vi "LP_Rx_and_BMon.vi"(0 "Rx":waveform(dbl)={"t0"=timestamp(3771075609.2144814 s since 1904-01-01), "dt"=4.999999999999579e-07, "Y"=array[336000 elements], "attributes"=variant("NI_ChannelName"=variant(string "H1/ai7"), "NI_UnitDescription"=variant(string "Volts"))}, 1 "Bias":waveform(dbl)={"t0"=timestamp(3771075609.3975773 s since 1904-01-01), "dt"=4.999999999999579e-07, "Y"=array[336000 elements], "attributes"=variant("NI_ChannelName"=variant(string "H1/ai5"), "NI_UnitDescription"=variant(string "Volts"))}, 2 "BMon":waveform(dbl)={"t0"=timestamp(3771075609.3975773 s since 1904-01-01), "dt"=4.999999999999579e-07, "Y"=array[336000 elements], "attributes"=variant("NI_ChannelName"=variant(string "H1/ai5"), "NI_UnitDescription"=variant(string "Volts"))}, 3 "BaselineSig":dbl[](array[numeric])=array[336000 elements]) -> (5 "RxBaselineSub":dbl[](graph), 6 "RX_Smooth":dbl[](array[numeric]), 7 "BiasSmooth":dbl[](array[numeric]), 8 "BMon Smooth":dbl[](array[numeric]), 9 "Bias Reconstructed":dbl[](array[numeric]))   [LabVIEW 2021]
uses:
  <vilib>/Analysis/baseanly.llb/Mean (DBL).vi
  <vilib>/Waveform/WDTOps.llb/WDT Number of Waveform Samples DBL.vi
  MPS_global_variables.vi
  <vilib>/measure/macond.llb/Continuous Waveform Convolution for 1 Chan.vi
  <vilib>/measure/matone.llb/Extract Single Tone Information 1 Chan.vi
  <vilib>/measure/NI_MAPro.lvlib
  <vilib>/Analysis/NI_AALBase.lvlib
  <vilib>/measure/NI_MABase.lvlib
panel:
  out "x/y":dbl=168000.0
  out "detected amplitude 2":dbl=0.10391083925713944 format="%.2p"
  out "Bias_IMon_Amps_MeanSub":waveform(dbl)(graph)={"t0"=timestamp(3771075609.3975773 s since 1904-01-01), "dt"=4.999999999999579e-07, "Y"=[], "attributes"=variant("NI_ChannelName"=variant(string "H1/ai5"), "NI_UnitDescription"=variant(string "Volts"))}
  in  "Bias Reconstruct Phase offset":dbl=-4.0 format="%#_13g"
  in  "index":i32
  out "BMon In":waveform(dbl)(graph)={"t0"=timestamp(3771075609.3975773 s since 1904-01-01), "dt"=4.999999999999579e-07, "Y"=array[336000 elements], "attributes"=variant("NI_ChannelName"=variant(string "H1/ai5"), "NI_UnitDescription"=variant(string "Volts"))}
  out "XY Graph":cluster{"Y":dbl[], "Y":dbl[]}[](graph)
  out "Bias_Reconstructed":dbl[](graph)
  out "BMon Smooth":dbl[](graph)
  out "Bias Smooth":dbl[](graph)
  out "Rx Smooth Graph":dbl[](graph)
  in  "advanced search":T1={"approx freq. (optional)"=-1.0, "search (+/- % of Fsampl.)"=5.0} {"search (+/- % of Fsampl.)" format="%0.2p"; "approx freq. (optional)" format="%0.2p"}
  in  "Crop Bias Periods":dbl=5.0
  out "Length_Conv":dbl=84.0
  out "Bias mT/V":dbl=249.6
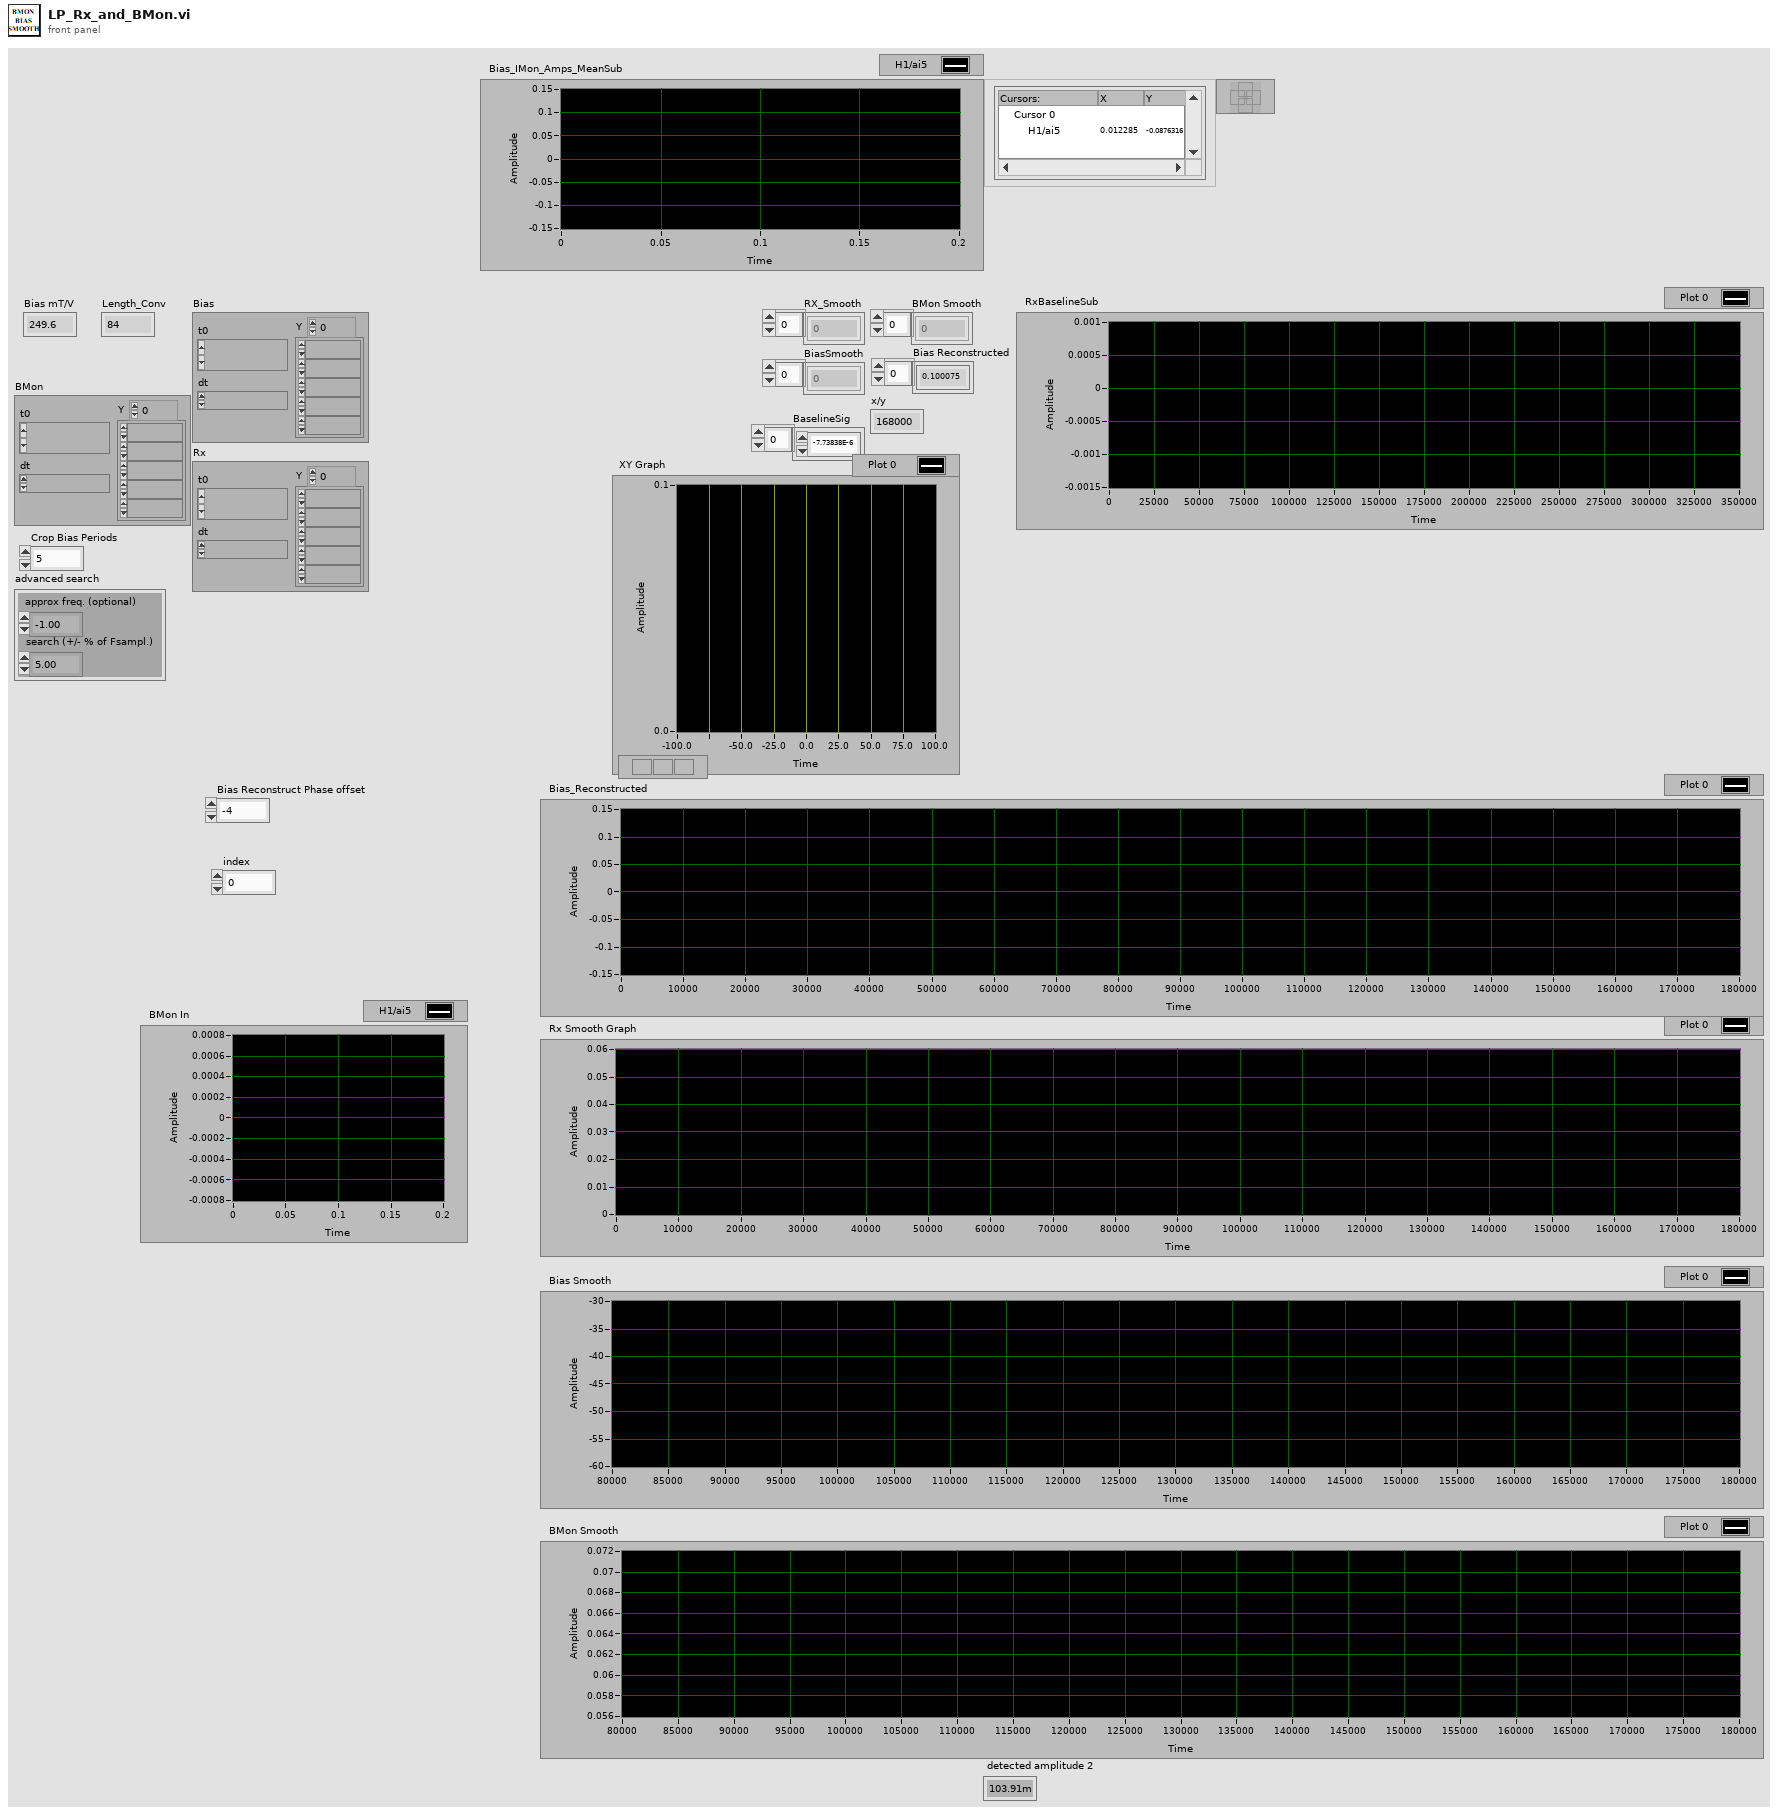
[diagram p1: front panel]
types:
  T1 = cluster{"approx freq. (optional)":dbl, "search (+/- % of Fsampl.)":dbl}
  T2 = cluster{"sample rate":dbl, "Tx freq":dbl, "Tx amp":dbl, "Tx cycles\nSpectroscopy":dbl, "Bias amp":dbl, "Bias freq":dbl, "Receive range":dbl, "Bias Periods\nMagnetometry":dbl, "Tx Freq Division Factor":dbl, "Drive Periods per Bias":dbl, "TX harmonics":dbl[]}
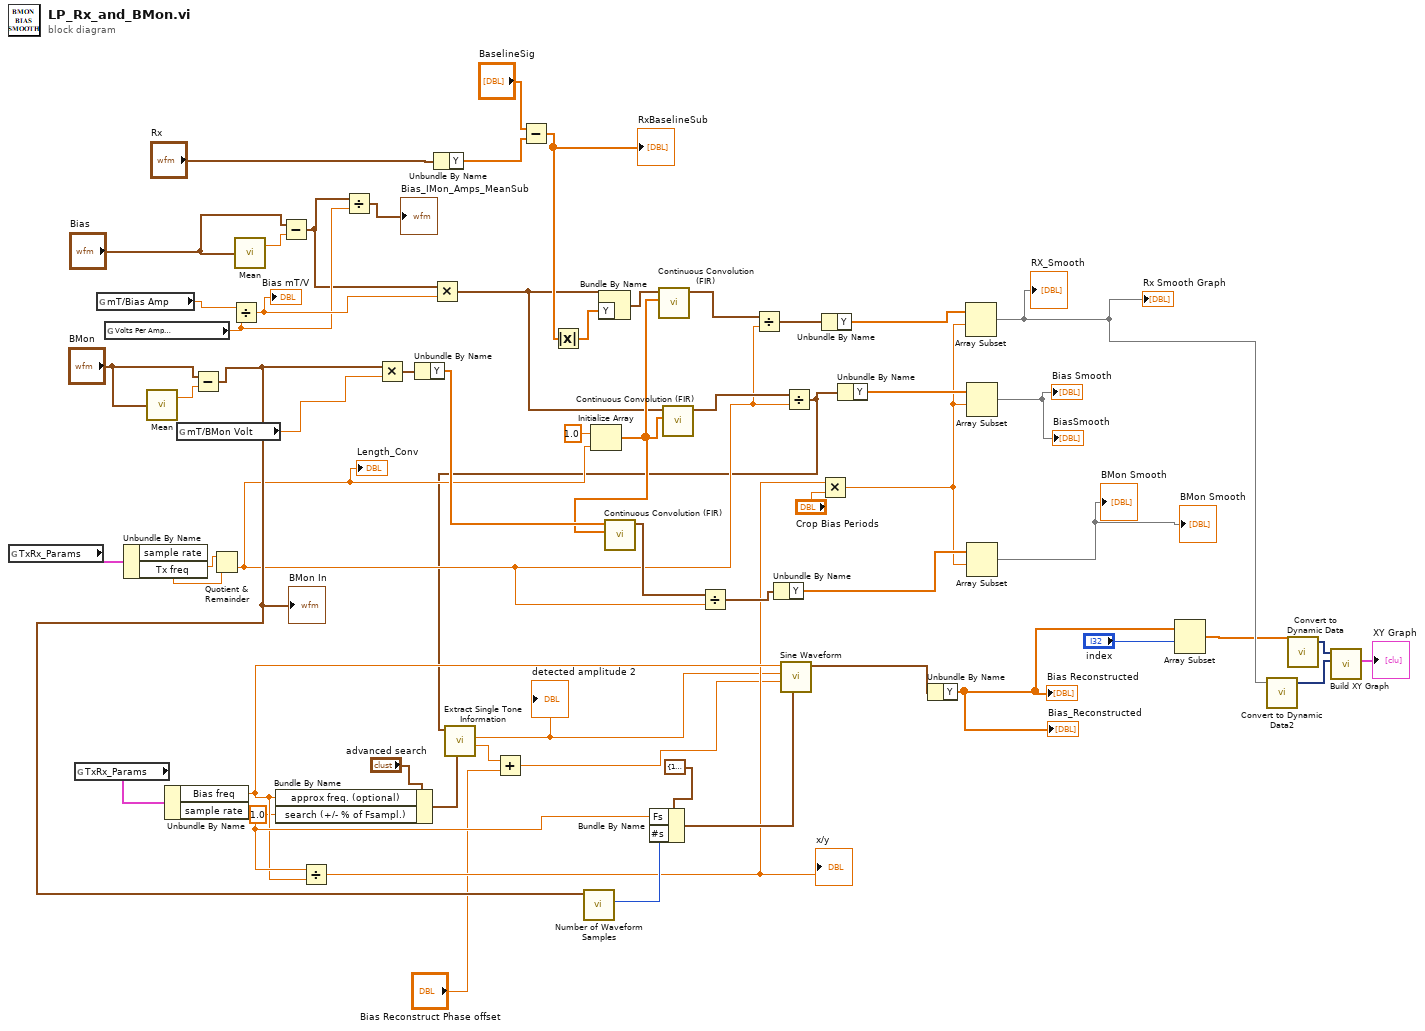
[diagram p0: block diagram]
diagram:
  n1 = global read "MPS_global_variables.vi" "TxRx_Params"() -> (w17:T2)
  n2 = global read "MPS_global_variables.vi" "TxRx_Params"() -> (w42:T2)
  n3 = global read "MPS_global_variables.vi" "mT/Bias Amp"() -> (w23:dbl)
  n4 = global read "MPS_global_variables.vi" "Volts Per Amp\nBias"() -> (w8:dbl)
  n5 = Unbundle By Name(w17) -> ("sample rate"=w15:dbl, "Tx freq"=w16:dbl)
  n6 = call-poly <vilib>:"Mean.vi"("X"="BMon") -> ("mean"=w45:dbl)  [unwired: 1 out]
  n7 = Unbundle By Name(w42) -> ("Bias freq"=w19:dbl, "sample rate"=w20:dbl)
  n8 = global read "MPS_global_variables.vi" "mT/BMon Volt"() -> (w22:dbl)
  n9 = Subtract(x="BMon", y=w45) -> (x-y=w31:waveform(dbl))
  "BMon In" <- w31
  n10 = Quotient & Remainder(x=w15, y=w16) -> (floor(x/y)=w14:dbl)  [unwired: 1 out]
  "Length_Conv" <- w14
  n11 = Divide(x=w23, y=w8) -> (x/y=w21:dbl)
  "Bias mT/V" <- w21
  n12 = call-poly <vilib>:"Mean.vi"("X"="Bias") -> ("mean"=w44:dbl)  [unwired: 1 out]
  n13 = Bundle By Name(cluster="advanced search", "approx freq. (optional)"=w19, "search (+/- % of Fsampl.)"=1.0) -> (w41:T1)
  n14 = Subtract(x="Bias", y=w44) -> (x-y=w7:waveform(dbl))
  n15 = Divide(x=w20, y=w19) -> (x/y=w18:dbl)
  "x/y" <- w18
  n16 = Divide(x=w7, y=w8) -> (x/y=→"Bias_IMon_Amps_MeanSub":waveform(dbl))
  n17 = Multiply(x=w31, y=w22) -> (x*y=w61:waveform(dbl))
  n18 = Unbundle By Name(w61) -> ("Y"=w52:dbl[])
  n19 = Multiply(x=w7, y=w21) -> (x*y=w3:waveform(dbl))
  n20 = Unbundle By Name("Rx") -> ("Y"=w25:dbl[])
  n21 = Subtract(x="BaselineSig", y=w25) -> (x-y=w24:dbl[])
  "RxBaselineSub" <- w24
  n22 = Absolute Value(x=w24) -> (abs(x)=w2:dbl[])
  n23 = call-poly <vilib>:"Number of Waveform Samples.vi"("waveform in"=w31) -> ("number of samples"=w36:i32)  [unwired: 8 in, 2 out]
  n24 = Initialize Array(1.0 ("element"), w14) -> (w51:dbl[])
  n25 = Bundle By Name(cluster=w3, "Y"=w2) -> (w1:waveform(dbl))
  n26 = call-poly <vilib>:"Continuous Convolution (FIR).vi"("kernel"=w51, "signal in"=w52) -> ("signal out"=w50:waveform(dbl))  [unwired: 8 in, 1 out]
  n27 = Bundle By Name(cluster=cluster{"Fs":dbl, "#s":dbl} {"Fs"=1000.0, "#s"=1000.0} ("sampling info"), "Fs"=w20, "#s"=w36) -> (w37:cluster{"Fs":dbl, "#s":dbl})
  n28 = call-poly <vilib>:"Continuous Convolution (FIR).vi"("kernel"=w51, "signal in"=w1) -> ("signal out"=w58:waveform(dbl))  [unwired: 8 in, 1 out]
  n29 = call-poly <vilib>:"Continuous Convolution (FIR).vi"("kernel"=w51, "signal in"=w3) -> ("signal out"=w57:waveform(dbl))  [unwired: 8 in, 1 out]
  n30 = Divide(x=w50, y=w14) -> (x/y=w49:waveform(dbl))
  n31 = Divide(x=w58, y=w14) -> (x/y=w59:waveform(dbl))
  n32 = Unbundle By Name(w49) -> ("Y"=w48:dbl[])
  n33 = Divide(x=w57, y=w14) -> (x/y=w4:waveform(dbl))
  n34 = call-poly <vilib>:"Extract Single Tone Information.vi"("advanced search"=w41, "time signal in"=w4) -> ("detected phase (deg)"=w13:dbl, "detected amplitude"=w5:dbl)  [unwired: 4 in, 4 out]
  "detected amplitude 2" <- w5
  n35 = Add(x=w13, y="Bias Reconstruct Phase offset") -> (x+y=w11:dbl)
  n36 = call <vilib>:"Sine Waveform.vi"("sampling info"=w37, "phase"=w11, "amplitude"=w5, "frequency"=w19) -> ("signal out"=w40:waveform(dbl))  [unwired: 6 in, 1 out]
  n37 = Multiply(x=w18, y="Crop Bias Periods") -> (x*y=w47:dbl)
  n38 = Unbundle By Name(w59) -> ("Y"=w56:dbl[])
  n39 = Unbundle By Name(w4) -> ("Y"=w54:dbl[])
  n40 = Unbundle By Name(w40) -> ("Y"=w27:dbl[])
  "Bias Reconstructed" <- w27
  "Bias_Reconstructed" <- w27
  n41 = Array Subset(array=w56, index=w47) -> (w32:dbl[])  [unwired: 1 in]
  "RX_Smooth" <- w32
  "Rx Smooth Graph" <- w32
  n42 = Array Subset(array=w54, index=w47) -> (→"BiasSmooth" →"Bias Smooth":dbl[])  [unwired: 1 in]
  n43 = Array Subset(array=w48, index=w47) -> (→"BMon Smooth" →"BMon Smooth":dbl[])  [unwired: 1 in]
  n44 = Array Subset(array=w27, index="index") -> (w29:dbl[])  [unwired: 1 in]
  n45 = call "Convert to Dynamic Data2"("Array"=w32) -> ("Dynamic Data Type"=w33:dynamicdata)  [unwired: 3 in]
  n46 = call "Convert to Dynamic Data"("Array"=w29) -> ("Dynamic Data Type"=w34:dynamicdata)  [unwired: 3 in]
  n47 = call "Build XY Graph"("Y Input"=w33, "X Input"=w34) -> ("XY Graph"=→"XY Graph":cluster{"X":dbl[], "Y":dbl[]}[])  [unwired: 8 in, 1 out]
